vi "Examples Stability Test.vi"() -> ()   [LabVIEW 2020, in "LcPictureBox.lvclass"]
uses:
  LcPictureBox.lvclass
  SmoothingMode.ctl
  Pen.ctl
  e1e9a9bd-98ff-476f-aab3-645122a4151d.vi
  <vilib>/numeric/Random Number (Range) DBL.vi
  d1ee4217-10e7-4f66-9caa-36ff55cbe2f3.vi
  System.Windows.Forms
panel:
  out "Interation1":i32
  in  "Stop":bool
  out "Interation2":i32
  out "Error Out":errorcluster[](array[cluster])
  in  "PictureBox":refnum<k24>(container)
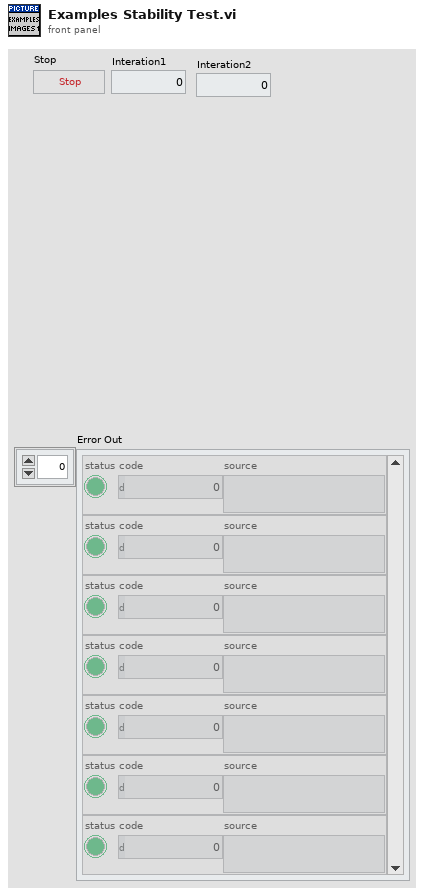
[diagram p1: front panel]
types:
  T1 = typedef "LcPictureBox.lvclass/Pen.ctl" = cluster{"Width":u16, "Style":enum32{"Solid", "Dash", "Dot", "DashDot", "DashDotDot"}}
  T2 = typedef "LcPictureBox.lvclass/SmoothingMode.ctl" = enum16{"None", "HighSpeed", "HighQuality", "AntiAlias"}
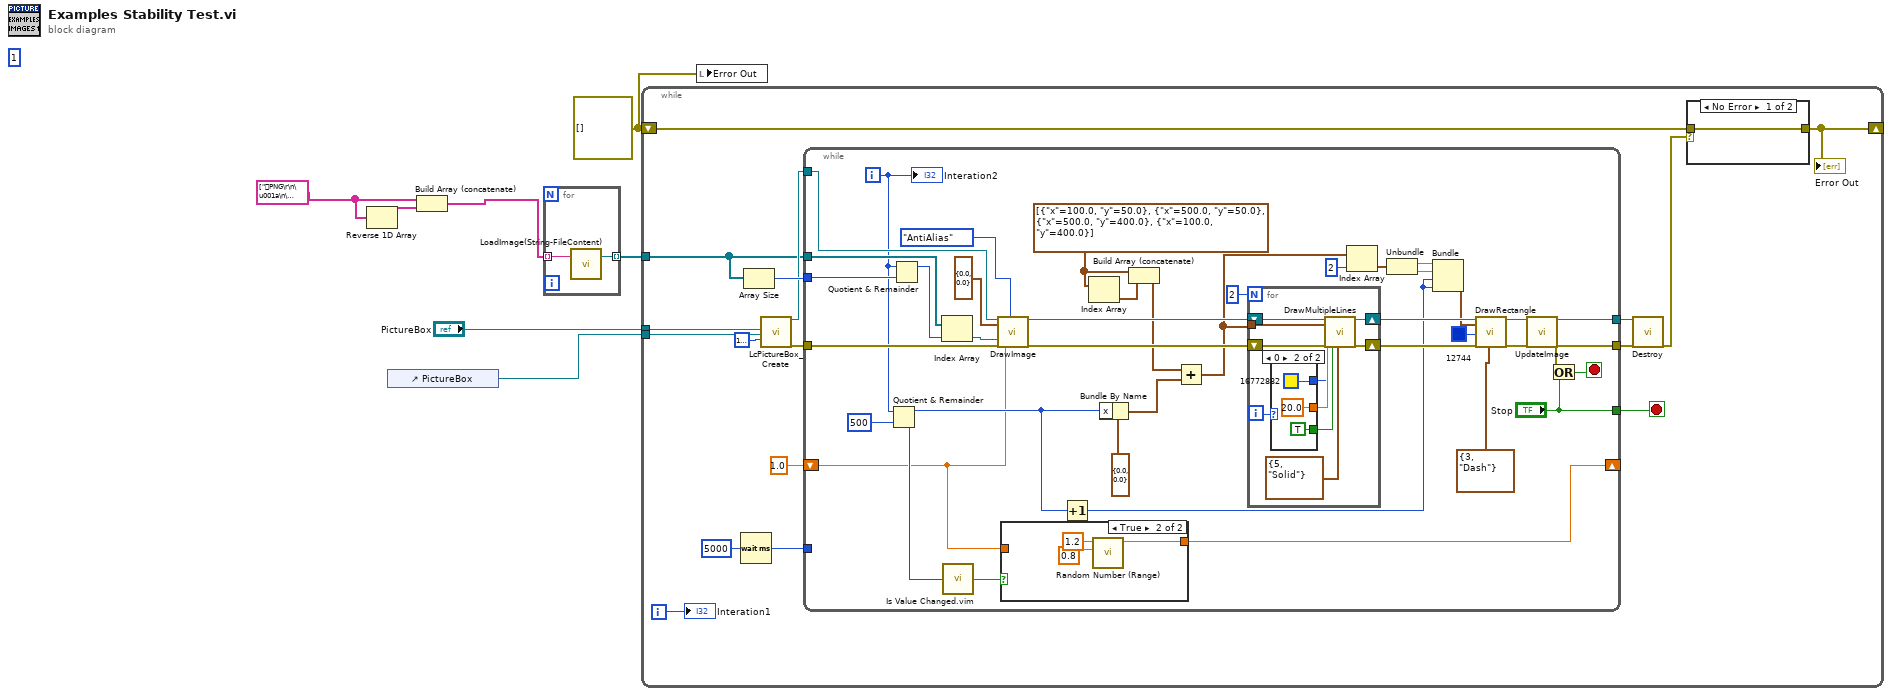
[diagram p0: block diagram]
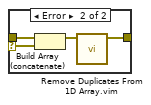
[diagram p2: hidden frame]
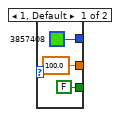
[diagram p4: hidden frame]
diagram:
  w1 = string[] ["PNG\r\n\u001a\n\u0000\u0000\u0000\rIHDR\u0000\u0000\u0004\\\u0000\u0000\u0002\b\u0002\u0000\u0000\u0000µ¦¹æ\u0000\u0000\u0000\u0006bKGD\u0000\u0000\u0000\u0000\u0000\u0000ùC»\u0000\u0000\u00006zTXtVersion\u0000\u0000x\u0001óK,ÉÌÏKÌQðÌ+.)*ÍMÍ+)Vðôu\fT\bË,\u0006Ê(Xèé\u0019\u0000\u0000\u0012y\fýZÐ|y\u0000\u0000\u0000\u000ftEXtNI Image Type\u00004ÉÁÏz\u0000\u0000 \u0000IDATx\u0001ì½\u0007X\u001bWÚþo÷¿ov³iNqbÇ+\u0018Lï½&$!¡$Ô\u0010¢*è½÷nlãÞ°Á»1îÆ½÷\u001a×¸÷n¾[L¢(É²ëlòf_gëÎ¹F3Ã\fç7÷ó<ç\u001dgG\u001fädçü½\\í5dëêüÜ\\ìÔR\u000fþ¤£¹»Ó/\u0012ÉÕÑÍÅ8´£­¦\u001cí­!\u0007;+;\u001b\u000bÈÆÚÜÚÊÌÒÜ\u0018²0327545621246Ô72Ð\u001b3rÖx=/\u000f¿´ô\u0002&G\u0014\u0014\u0016\u001b\u0015*\u000eð\u0017J¥aá1ñ<±, 0X\u0012\"\u0017ÉÂE²ÐÀ aPª#\u000bñðe0ø\u0001Þ~LqH\u0018FìÝÜC¢b\u0018\\¾$4Îá9<¤!r\u000e_\"\u0004{}¿\u001c®õ÷\u000fF|òé\u0004\u001f\u001fÙ¶-§6m>±¾÷ðªu{º×îíX³gNçÖ¹+wv÷Z¶ýÈÆÃgrêlÝ=\u0002#£¢þB,\"8£¸$)¿0¿¢êÞËWÐýþ~èAÿ/o<{vóùó+\u000f\u001f^ú\u0014í\u001b7ö<½rË¶Ùí\u001dÓ\u0017·u¬íYÞ³ióÞ\u0003GÎ_<yéúów\u001e>Ù¹nãÌ%Í\u000b,\\¾zï©ów½zÜßÿ...", "PNG\r\n\u001a\n\u0000\u0000\u0000\rIHDR\u0000\u0000\u0004\\\u0000\u0000\u0002\b\u0002\u0000\u0000\u0000µ¦¹æ\u0000\u0000\u0000\u0006bKGD\u0000\u0000\u0000\u0000\u0000\u0000ùC»\u0000\u0000\u00006zTXtVersion\u0000\u0000x\u0001óK,ÉÌÏKÌQðÌ+.)*ÍMÍ+)Vðôu\fT\bË,\u0006Ê(Xèé\u0019\u0000\u0000\u0012y\fýZÐ|y\u0000\u0000\u0000\u000ftEXtNI Image Type\u00004ÉÁÏz\u0000\u0000 \u0000IDATx\u0001ì½\u0005x\u001bWÚþÝo÷¿ow»¥¤mÚ$mÃ\u001d33Ë$K²d%YdIF\u0019eÌÌ!\u001cr\u0012ÇíÄap9i°aæø»åiUµ]ï¦Û¾Ý7Ýôº{®££ÑÌxF±ÏoîçyÎ;®ÎN?ÈÅÁõ{¹»:êÈÞÝõ;y¸9h¥\u001düIGw\u001bO\u000f_$»³\u0013qh\u0017g{]9;ÚBN\u000e6\u000evV­¥­µ¥)deabinlnjbfbljlhbd0â«/õÆè\u0019màã\u0015^ÀädáqÑ\t©âÈ@¡T\u001a\u001e\u0015\u0011À\u0013ËC$¡\n<B$\u000f\u000b\n\te¡<ÔËÁà\u0007ù\u00060Å¡á\u0018qôð\fepù°\b:çDò*8|@\u0012âEöÿbÈ¿ðåÀOÆùùÉ·n>µqÓµ=W¬ÙÓ½zoÇª=³:·Ì^¾³{Ç©%Ûl8|&§n¢½§WpTtt²*P(Gd\u0014$ç\u0017æWTÝ{ù\nºßÛ\u000b=èí½óòågÏn>~åáÃëO¢=sãÆ§oÞÚÜÞ1ma[ÇêuK×mÜ´÷Àó\u0017O^º~äüåOv®Ù0cQgÓüEó®Ü{êüÝg¯\u001e÷ö...", "PNG\r\n\u001a\n\u0000\u0000\u0000\rIHDR\u0000\u0000\u0004\\\u0000\u0000\u0002\b\u0002\u0000\u0000\u0000µ¦¹æ\u0000\u0000\u0000\u0006bKGD\u0000\u0000\u0000\u0000\u0000\u0000ùC»\u0000\u0000\u00006zTXtVersion\u0000\u0000x\u0001óK,ÉÌÏKÌQðÌ+.)*ÍMÍ+)Vðôu\fT\bË,\u0006Ê(Xèé\u0019\u0000\u0000\u0012y\fýZÐ|y\u0000\u0000\u0000\u000ftEXtNI Image Type\u00004ÉÁÏz\u0000\u0000 \u0000IDATx\u0001ì½\u0007X\u001bWÚþo÷¿ov³iNqb§¸bé½wÑ$$T\u001aBTQE\u0011½÷ÞÝpÃ\rÛ\u0018\fØØ`c{ï½Ûq{ïæ»Å$,»Î&oöuÖ¹îëèh43ÌÈp~s?ÏsÞrr°ÿA¶NßËÅÉNC6.NßÉÕÙV-õàO:Û¸¹:þ\"\\\u001c\\íC;:ØhÊÁÎ\n²·µ´µ6¬­Ì¬,M-Ì sSC3\u0013\u0003cC\u0003\u0013#C´\u0006zÆ|õ¥¶¶Öx]OwßÔ´|&G\u0014\u0018\u001a\u0013\u0019\"\u000e\n÷\u0013J¥¡\u0011aÑq<±Ì? H\u0012,\u0017ÉÂD²\u0010ÿ@a`°ª#\u000bv÷a0øþ^¾Lqp(Fì\\Ý#£\u0019\\¾$$ÎáÙÜ¥Ár\u000e_\"\u0004¹}>\u001f©õ÷÷¾üèãÞÞ²-NnØx|mÿ¡îÞÝ]kö´¯Þ=·có¼U;º¶\\¾õðúC§³k§Ø¸¹\u0007DDF&*ý\u0012YxPzQqb^A^yåÝ\u0017/¡{\u0003\u0003ÐýÛ/^\\úôÆ³g\u001f<¸öä\tÚÓ×¯ï>qjÕ¦-Mmí3´¶¯é[Ñ·aãýÏ]8qñÚásv\u001c:ÑÑ»~öÒÆEK\u0017­èÙsòÜ§/\u001f\r\f<Æ...", "PNG\r\n\u001a\n\u0000\u0000\u0000\rIHDR\u0000\u0000\u0004\\\u0000\u0000\u0002\b\u0002\u0000\u0000\u0000µ¦¹æ\u0000\u0000\u0000\u0006bKGD\u0000\u0000\u0000\u0000\u0000\u0000ùC»\u0000\u0000\u00006zTXtVersion\u0000\u0000x\u0001óK,ÉÌÏKÌQðÌ+.)*ÍMÍ+)Vðôu\fT\bË,\u0006Ê(Xèé\u0019\u0000\u0000\u0012y\fýZÐ|y\u0000\u0000\u0000\u000ftEXtNI Image Type\u00004ÉÁÏz\u0000\u0000 \u0000IDATx\u0001ì\u0007x\u0013WÚ¶óßîf7J*!\t¡ØØ¸÷Þå&K²duYÍ²\\å*\u0017É½÷^1`©\u0006\r\u0018\f\u0018\fÞ;Þkè½ãÿ\u0011(Jñ.ÙäËn²äzr®ÑÑhftFÈçÖó¾ïyÍÝÕå;¹9¹+Owg\u001d9zº#/\u000f'­´?ØÐÝÇÛËígäéêåáBÚÍÕQW®Îö\rä`omogekm\u000eÙXY[Z}§/?\u001bf¨?V_ÏØ×QÄfå\tñÊtIX4W$EÆDÅ'ñ%òà0i¸B,\u0012Ë#D¡áP\u0016\u0016,\u000f÷\td0\u0004ÁþAL<D§³wD\\\u0002Ã\u000fa\tnÞ~¡\u00111PAq%G ýdØ¨7Þ\u001cúÎ{£üü¥6\u001c[»öðÊ5û÷íì^µkÑÊÝ3\u0017n³l{ÏÖc7\u001f\\{àD^C£·OHLllª+Ê£Ã²JËR\u000b\u000b«jn?{\u000eÝ\u0019\u0018î\u000e\fÜ|öìêãÇ×<¹xïÞGÐ¸zuçÑãË6lÖµpò¼Î+W/Y½ný®½\u0007O;zþÊÁÓ\u0017¶\u001d8º¨oíÔùZçÌ³¤w×±Ó·\u001e?00ð\u0010\u0007|öôÎÀ3ÍÁk...", "PNG\r\n\u001a\n\u0000\u0000\u0000\rIHDR\u0000\u0000\u0004\\\u0000\u0000\u0002\b\u0002\u0000\u0000\u0000µ¦¹æ\u0000\u0000\u0000\u0006bKGD\u0000\u0000\u0000\u0000\u0000\u0000ùC»\u0000\u0000\u00006zTXtVersion\u0000\u0000x\u0001óK,ÉÌÏKÌQðÌ+.)*ÍMÍ+)Vðôu\fT\bË,\u0006Ê(Xèé\u0019\u0000\u0000\u0012y\fýZÐ|y\u0000\u0000\u0000\u000ftEXtNI Image Type\u00004ÉÁÏz\u0000\u0000 \u0000IDATx\u0001ì\u0007x\u0013WÚ¶óßîf7J*PllÜ{ïU²$KV±$«Y«\\å\"¹÷Þ+\u0006L1½\u0018\u001bc0`0`Lï½÷\u001azïíäI\u0014¥xCv³Ù/Yr=9×èh43:#äsëyß÷¼áêìô\\\u001c\\¿»«£ìÝ]¿FÎ\u001flhïãåáòäéîìáæDÚÅÙ^[Î¶\u0015dgkikcami\nYYX\u001b|§¯>\u001f®¯;NWÇÐÇ^Èfd\u0011ñq4qhT P*KäeAÁ¡0¹H\u0016)\u000bCÂ 44H\u0016æíÏ`ðH\u0001L<D§£Wxl<Ã\u000bfñ\u0005.^¾!áÑP~Q\u0005/ùløè·Þ\u001eúÞ\u0007£}IM\u001b¯[wdÕÚ}+zwv­ÞµxÕîY\u001bç-ßÞ½õøÍ\u0007×\u001d8[ßlïå\u001d\u001c\u001d\u0013¢\f\u0014JdQ¡%¥)\u0005E\u0005Õw¿î¾|\tÝ{ùòÖóç×<¹þôé¥û÷¯>~öäµk;X¾aÓôÎ)\u000bÚ;W­Yº¦ý®½\u0007Ï?váêÁ3\u0017·\u001d8¶¸wÝ´[æ-·´g×ñ3·¼xøòå#\u001cðù³»/«\u000fþB..."]
  w4 = errorcluster[] []
  (unwired) 1
  n1 = Reverse 1D Array(array=w1) -> (reversed array=w2:string[])
  n2 = control-ref of="PictureBox"() -> (w3:refnum<vi>)
  n3 = Build Array (concatenate)(w1, w2) -> (w6:string[])
  n4 = for {
    tunnel: w6 -> [w9] mode=indexing
    tunnel: [w8] -> w5 mode=indexing
    n5 = call "LoadImage(String-FileContent).vi"("ImageFileContent"=w9) -> ("ImageOut"=w8:refnum<k24>)  [unwired: 16 in, 2 out]
  }
  n6 = while {
    tunnel: "PictureBox" -> [w26]
    tunnel: w5 -> [w21]
    shift-right: [w13] -> _
    shift-left: w4 -> [w15]
    tunnel: w3 -> [w10]
    i -> [w16]
    stop <- w17 stop-if-true
    n7 = Wait (ms)(milliseconds to wait=u32 5000) -> (millisecond timer value=w12:u32)
    n8 = Array Size(array=w21) -> (size(s)=w24:i32)
    n9 = call "LcPictureBox_Create.vi"("PictureBox"=w26, "PictureBoxActiveXReference"=w10, "BgColor(None)"=u32 16777216) -> ("reference out"=w23:refnum<class "LcPictureBox.lvclass">, "Error Out"=w22:errorcluster)  [unwired: 14 in, 1 out]
    n10 = while {
      tunnel: w24 -> [w70]
      tunnel: w23 -> [w69]
      tunnel: w22 -> [w68]
      tunnel: w21 -> [w67]
      tunnel: [w64] -> w20
      tunnel: [w52] -> w19
      shift-right: [w34] -> _
      shift-left: 1.0 ("x") -> [w35]
      tunnel: ["Stop"] -> w17
      tunnel: w12 -> [_]
      i -> [w32]
      stop <- w51 stop-if-true
      w58 = cluster{"x":dbl, "y":dbl}[] [{"x"=100.0, "y"=50.0}, {"x"=500.0, "y"=50.0}, {"x"=500.0, "y"=400.0}, {"x"=100.0, "y"=400.0}] ("LineEndPoints")
      n11 = Quotient & Remainder(x=w32, y=500) -> (x-y*floor(x/y)=w42:i32, floor(x/y)=w37:i32)
      n12 = Quotient & Remainder(x=w32, y=w70) -> (x-y*floor(x/y)=w66:i32)  [unwired: 1 out]
      n13 = Index Array(array=w67, index=w66) -> (element=w65:refnum<k24>)
      n14 = call "Is Value Changed.vim"("value"=w37) -> ("changed or first call?"=w36:bool)
      n15 = call-dynamic "DrawImage.vi"("reference in"=w69, "UpperLeftCorner(0,0)"=cluster{"x":sgl, "y":sgl} {"x"=0.0, "y"=0.0} ("UpperLeftCorner"), "Image"=w65, "Error In"=w68, "ScaleFactor(1)"=w35, "SmoothingMode(AntiAlias)"=SmoothingMode."AntiAlias" ("SmoothingMode")) -> ("reference out"=w62:refnum<class "LcPictureBox.lvclass">, "Error Out"=w61:errorcluster)  [unwired: 12 in]
      n16 = case shown="True" w36 {
        tunnel: w35 -> [w72 _]
        tunnel: [w72 w73] -> w34
        frame False {
        }
        frame True {
          n17 = call-poly <vilib>:"Random Number (Range).vi"("lower bound (0)"=0.8 ("upper bound (100)"), "upper bound (100)"=1.2) -> ("number"=w73:dbl)  [unwired: 9 in]
        }
      }
      n18 = Increment(x=w42) -> (x+1=w41:i32)
      n19 = Index Array(array=w58) -> (element=w57:cluster{"x":dbl, "y":dbl})  [unwired: 1 in]
      n20 = Bundle By Name(cluster=cluster{"x":dbl, "y":dbl} {"x"=0.0, "y"=0.0} ("Point"), "x"=w42) -> (w54:cluster{"x":dbl, "y":dbl})
      n21 = Build Array (concatenate)(w58, w57) -> (w53:cluster{"x":dbl, "y":dbl}[])
      n22 = Add(x=w53, y=w54) -> (x+y=w47:cluster{"x":dbl, "y":dbl}[])
      n23 = for {
        N: 2 -> [_]
        tunnel: w47 -> [w81]
        shift-right: [w83] -> w49
        shift-left: w62 -> [w85]
        shift-right: [w82] -> w60
        shift-left: w61 -> [w84]
        i -> [w76]
        n24 = case shown="0" w76 {
          tunnel: [FALSE ("Fill(False)") TRUE ("Fill(False)")] -> w79
          tunnel: [100.0 ("Alpha(100%)") 20.0 ("Alpha(100%)")] -> w78
          tunnel: [u32 3857408 ("Color(Black)") u32 16772882 ("Color(Black)")] -> w77
          frame 1, Default {
          }
          frame 0 {
          }
        }
        n25 = call-dynamic "DrawMultipleLines.vi"("reference in"=w85, "LineEndPoints"=w81, "Color(Black)"=w77, "Alpha(100%)"=w78, "Error In"=w84, "Fill(False)"=w79, "Pen(Width=1, Solid)"=T1 {"Width"=5, "Style"=enum."Solid"}) -> ("reference out"=w83:refnum<class "LcPictureBox.lvclass">, "Error Out"=w82:errorcluster)  [unwired: 11 in]
      }
      n26 = Index Array(array=w47, index=2) -> (element=w45:cluster{"x":dbl, "y":dbl})
      n27 = Unbundle(w45) -> ("x"=w44:dbl, "y"=w43:dbl)
      n28 = Bundle("x"=w44, "y"=w43, w41, w41) -> (w40:cluster{"x":dbl, "y":dbl, i32, i32})  [unwired: 1 in]
      n29 = call-dynamic "DrawRectangle.vi"("reference in"=w49, "Rectangle"=w40, "Color(Black)"=u32 12744, "Error In"=w60, "Pen(Width=1, Solid)"=T1 {"Width"=3, "Style"=enum."Dash"}) -> ("reference out"=w48:refnum<class "LcPictureBox.lvclass">, "Error Out"=w50:errorcluster)  [unwired: 13 in]
      n30 = call-dynamic "UpdateImage.vi"("reference in"=w48, "Error In"=w50) -> ("reference out"=w64:refnum<class "LcPictureBox.lvclass">, "Error Out"=w52:errorcluster)  [unwired: 14 in, 2 out]
      n31 = Or(x=w52, y="Stop") -> (x .or. y?=w51:bool)
      "Interation2" <- w32
    }
    n32 = call-dynamic "Destroy.vi"("reference in"=w20, "Error In"=w19) -> ("Error Out"=w14:errorcluster)  [unwired: 16 in, 1 out]
    n33 = case shown="No Error" w14 {
      selector: w14 -> [_ w30]
      tunnel: w15 -> [w27 w31]
      tunnel: [w27 w28] -> w13
      frame No Error {
      }
      frame Error {
        n34 = Build Array (concatenate)(w31, w30) -> (w29:errorcluster[])
        n35 = call "Remove Duplicates From 1D Array.vim"("array"=w29) -> ("array with duplicates removed"=w28:errorcluster[])  [unwired: 10 in]
      }
    }
    "Error Out" <- w13
    "Interation1" <- w16
  }
  n36 = local write "Error Out"(w4) -> ()
